vi "EchoSpacing2.vi"() -> ()   [LabVIEW 2016]
uses:
  <vilib>/Analysis/3filter.llb/Filter Passband Type.ctl
  <vilib>/Analysis/NI_AALBase.lvlib
  <vilib>/Analysis/NI_AAL_SigProc.lvlib
  <vilib>/measure/NI_MABase.lvlib
panel:
  out "x/y 2":waveform(dbl)(graph)
  out "output waveform 4":waveform(dbl)(graph)
  out "output waveform 3":waveform(dbl)(graph)
  out "x after average":waveform(dbl)(graph)
  out "output waveform 2":waveform(dbl)(graph)
  out "Change in Speed of Sound":waveform(dbl)(graph)
  out "Phase":waveform(dbl)(graph)={"t0"=timestamp(0 s since 1904-01-01), "dt"=0.01, "Y"=[0.24211856243178442, 0.2979552577953536, 0.11762633618423823, -2.123508525918916, 0.20375659578318772, 0.23633325543017147, 0.10596858427793898, 0.35715128699234333, 0.3077330737862175, 0.29550230623359586, 0.26625637959678994, 0.4264526096514324]}
  out "millisecond timer value":u32=1848068
  out "Array":dbl[](array[numeric])=[0.6752734595800559, 1.1017260692314883, 0.6444600524294382, -1.442367499041461, -0.42475301826616657, 0.660304709391192, -1.2354533445502307, 0.27782180017105296, 1.2450593883598915, -0.8212746442960503, 0.8254110535070931, -0.826966642108493, 0.9668932937884392, -0.35218129117363, -0.35017284449625363, -1.426552428665809, 1.4327256876579455, 0.8973316502630515, 0.47447322742299236, -0.049748678045329967, 0.1127488236132522, -0.9412473014471964]
  out "initialized array":dbl[](array[numeric])
  out "Time Locations":dbl[](array[numeric])=[7.954456871737136e-07, 1.0829944804064152e-06, 1.2197668992928399e-06, 2.066421151225249e-06, 3.3334485136545128e-06, 4.592995774084014e-06, 5.857096715588158e-06, 7.158942345651641e-06, 8.398045018304592e-06, 9.645253296365048e-06, 1.090845897308631e-05, 1.2214698983664545e-05, 1.345038714346347e-05, 1.4701419228763196e-05, 1.4750655022908824e-05, 1.5970949694343346e-05, 1.6041105911005864e-05, 1.7231158138687473e-05, 1.7298645289114775e-05, 1.7383164294270303e-05, 1.8517816256101673e-05, 1.9782665116356317e-05]
  in  "Continuous":bool=TRUE
  in  "Run":bool
  out "output waveform 5":waveform(dbl)(graph)={"t0"=timestamp(0 s since 1904-01-01), "dt"=4e-10, "Y"=array[100000 elements]}
  out "Waveforms":waveform(dbl)[](graph)=[{"t0"=timestamp(0 s since 1904-01-01), "dt"=4e-10, "Y"=array[100000 elements]}, {"t0"=timestamp(2.599999999999738e-07 s since 1904-01-01), "dt"=4e-10, "Y"=array[100000 elements]}]
  out "output waveform":waveform(dbl)(graph)={"t0"=timestamp(2.599999999999738e-07 s since 1904-01-01), "dt"=4e-10, "Y"=array[100000 elements]}
  in  "frequency":dbl=220.0 format="%0.2p"
  in  "Channel (0: Channel 1)":u16(ring) items=["Channel 1", "Channel 2", "Channel 3", "Channel 4", "Math", "Reference 1", "Reference 2", "Reference 3", "Reference 4", "D0", "D1", "D2", "D3", "D4", "D5", "D6", "D7", "D8", "D9", "D10", "D11", "D12", "D13", "D14", "D15", "Amplitude", "Frequency", "Phase", "Normal", "Average", "Maximum Peak Hold", "Minimum Peak Hold"]
  in  "VISA Resource Name":refnum<visa-resource-name>="TCPIP0::10.84.241.74::inst0::INSTR"
  out "Waveform":waveform(dbl)(graph)={"t0"=timestamp(0 s since 1904-01-01), "dt"=4e-10, "Y"=array[100000 elements]}
  in  "threshold":dbl=0.05 format="%0.2f"
  in  "width":i32=150 min=3
  in  "low cutoff freq: fl":dbl=20.0 format="%0.4f"
  out "error":i32
  in  "order":i32=3
  out "total time":u32=34
  # "Single"
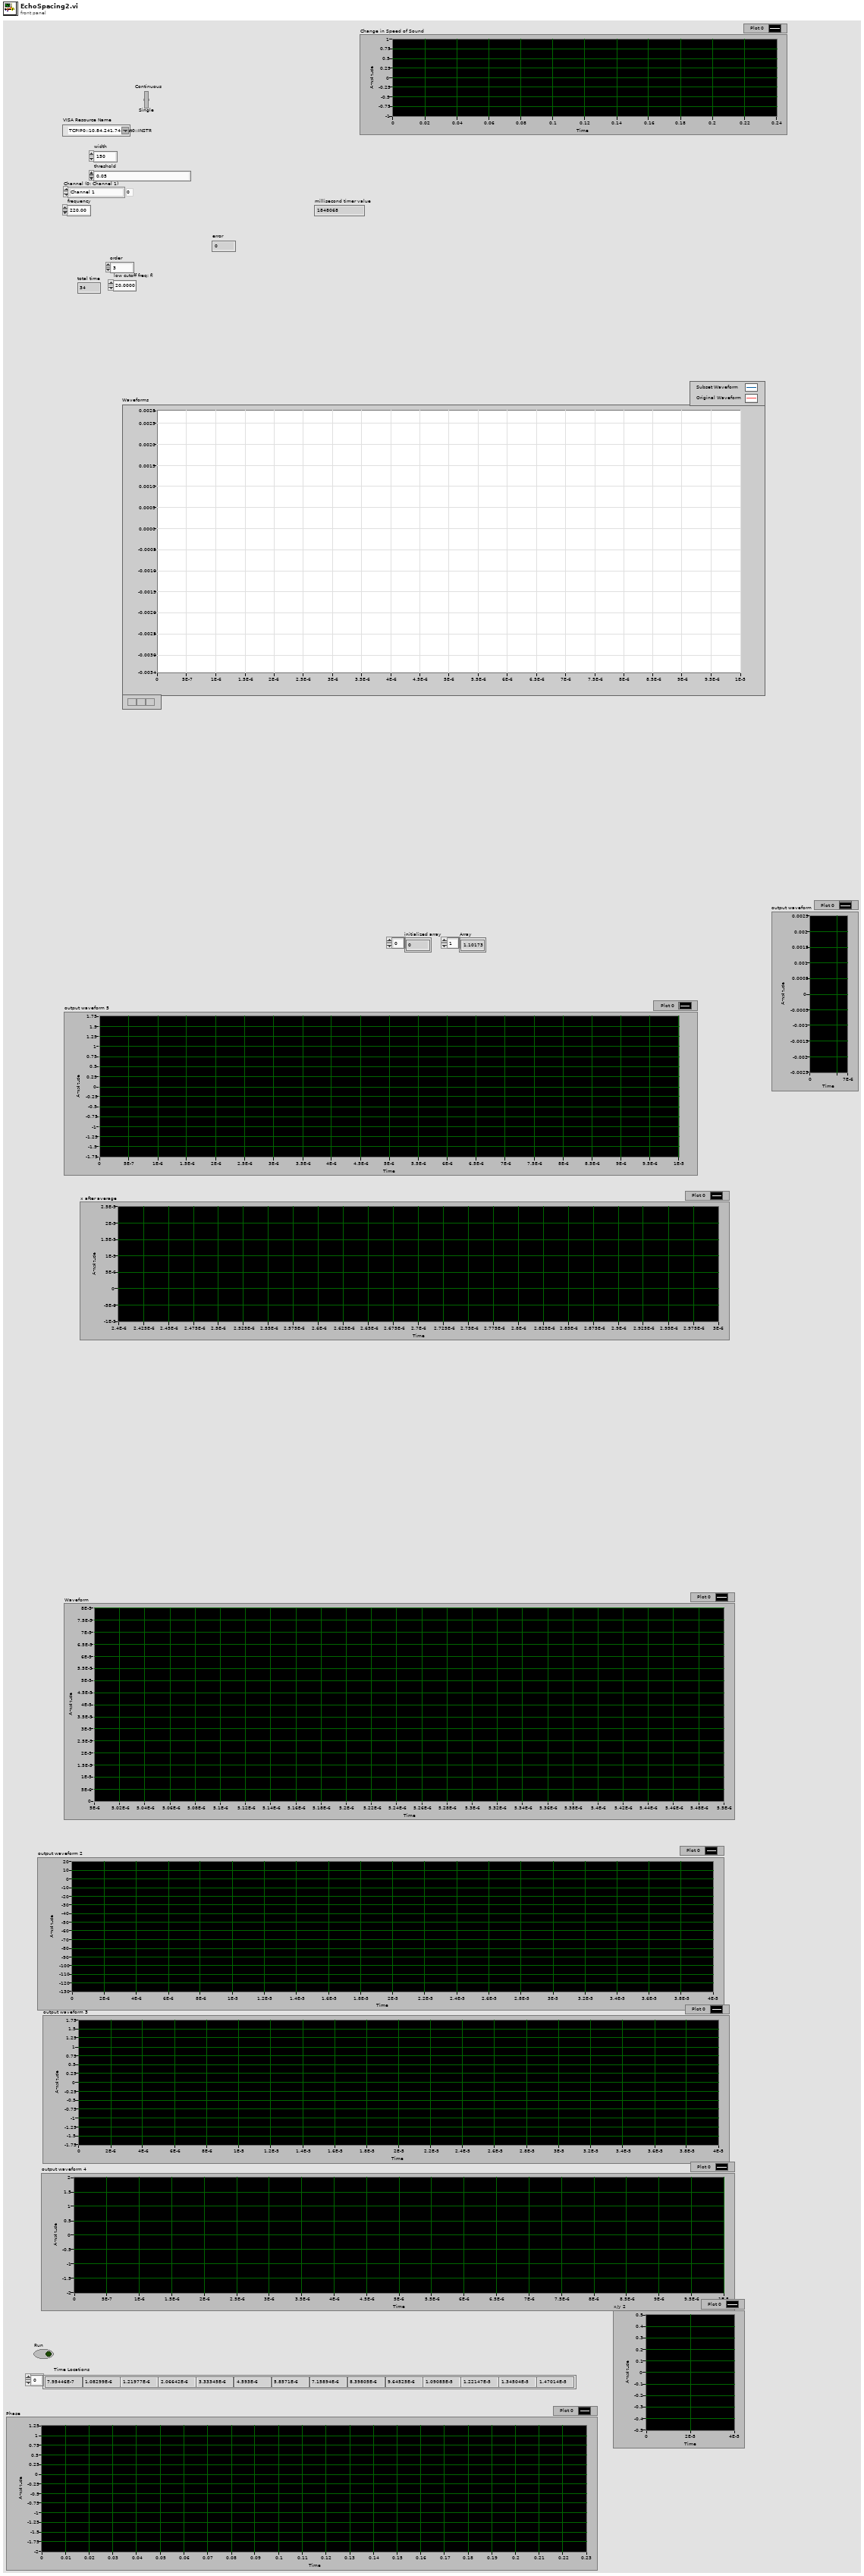
[diagram p1: front panel]
types:
  T1 = typedef "NI_AALBase.lvlib/Filter Passband Type.ctl" = enum32{"Lowpass", "Highpass", "Bandpass", "Bandstop"}
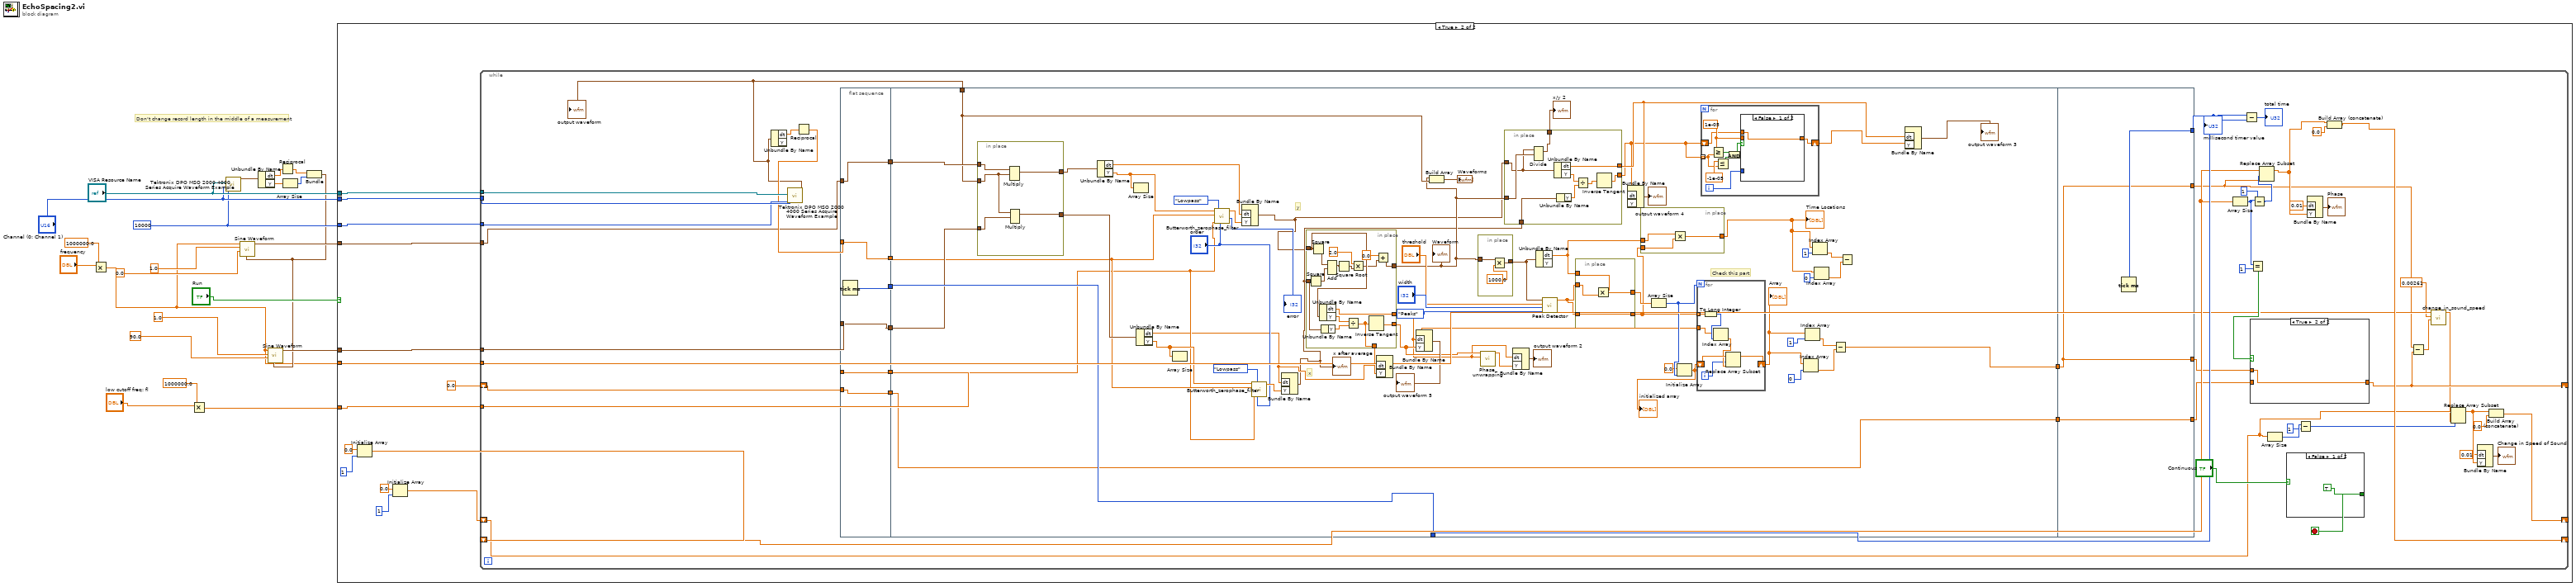
[diagram p0: block diagram]
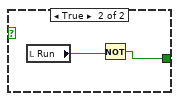
[diagram p4: hidden frame]
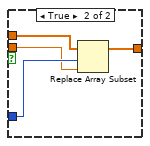
[diagram p5: hidden frame]
diagram:
  w14 = u32 10000 ("Maximum Time (10000ms)")
  # "Don't change record length in the middle of a measurement"
  n1 = Multiply(x="frequency", y=1000000.0) -> (x*y=w1:dbl)
  n2 = Multiply(x="low cutoff freq: fl", y=1000000.0) -> (x*y=w18:dbl)
  n3 = call "Tektronix DPO MSO 2000 4000 Series Acquire Waveform Example.vi"("Maximum Time (10000ms)"=w14, "Channel (0: Channel 1)"="Channel (0: Channel 1)", "VISA Resource Name"="VISA Resource Name") -> ("output waveform"=w7:waveform(dbl))  [unwired: 8 in]
  n4 = Unbundle By Name(w7) -> ("dt"=w5:dbl, "Y"=w6:dbl[])
  n5 = Reciprocal(x=w5) -> (1/x=w4:dbl)
  n6 = Array Size(array=w6) -> (size(s)=w3:i32)
  n7 = Bundle(w4, w3) -> (w2:cluster{dbl, i32})  [unwired: 1 in]
  n8 = call <vilib>:"Sine Waveform.vi"("sampling info"=w2, "phase"=0.0, "amplitude"=1.0, "frequency"=w1) -> ("signal out"=w8:waveform(dbl))  [unwired: 6 in, 1 out]
  n9 = call <vilib>:"Sine Waveform.vi"("sampling info"=w2, "phase"=90.0, "amplitude"=1.0, "frequency"=w1) -> ("signal out"=w11:waveform(dbl))  [unwired: 6 in, 1 out]
  n10 = case shown="True" "Run" {
    tunnel: "VISA Resource Name" -> [_ w36]
    tunnel: "Channel (0: Channel 1)" -> [_ w35]
    tunnel: w14 -> [_ w34]
    tunnel: w18 -> [_ w33]
    tunnel: w11 -> [_ w29]
    tunnel: w8 -> [_ w28]
    tunnel: w1 -> [_ w26]
    frame False {
    }
    frame True {
      n11 = Initialize Array(0.0 ("element"), 1 ("dimension size")) -> (w30:dbl[])
      n12 = Initialize Array(0.0 ("element"), 1 ("dimension size")) -> (w23:dbl[])
      n13 = while {
        tunnel: w36 -> [w79]
        tunnel: w35 -> [w78]
        tunnel: w34 -> [w77]
        tunnel: w33 -> [w75]
        shift-right: [w63] -> _
        shift-left: w30 -> [w70]
        tunnel: w29 -> [w67]
        tunnel: w28 -> [w66]
        shift-right: [w52] -> _
        shift-left: 0.0 -> [w55]
        tunnel: w26 -> [w53]
        shift-right: [w42] -> _
        shift-left: w23 -> [w45]
        stop <- w73 stop-if-true
        n14 = call "Tektronix DPO MSO 2000 4000 Series Acquire Waveform Example.vi"("Maximum Time (10000ms)"=w77, "Channel (0: Channel 1)"=w78, "VISA Resource Name"=w79) -> ("output waveform"=w37:waveform(dbl))  [unwired: 8 in]
        "output waveform" <- w37
        n15 = Unbundle By Name(w37) -> ("dt"=w38:dbl)  [unwired: 1 out]
        n16 = Reciprocal(x=w38) -> (1/x=w76:dbl)
        n17 = flat-sequence {
          tunnel: [w98] -> w87
          tunnel: w76 -> [w97]
          tunnel: [w97] -> w86
          tunnel: [w96] -> w85
          tunnel: w67 -> [w96]
          tunnel: w66 -> [w95]
          tunnel: [w95] -> w84
          tunnel: w75 -> [w94]
          tunnel: [w94] -> w83
          tunnel: w55 -> [w93]
          tunnel: [w93] -> w58
          tunnel: [w155] -> w81
          tunnel: w87 -> [w155]
          tunnel: w86 -> [w137]
          tunnel: w85 -> [w151]
          tunnel: w37 -> [w135]
          tunnel: w84 -> [w152]
          tunnel: w83 -> [w136]
          tunnel: [w99] -> w72
          tunnel: w58 -> [w116]
          tunnel: [w116] -> w57
          tunnel: [w218] -> w82
          tunnel: w72 -> [w216]
          tunnel: [w216] -> w51
          tunnel: w57 -> [w217]
          tunnel: [w217] -> w56
          tunnel: [w216] -> w54
          frame #0 {
            n18 = Tick Count (ms)() -> (millisecond timer value=w98:u32)
          }
          frame #1 {
            # "Check this part"
            # "x"
            # "y"
            n19 = in-place {
              in-place-border: w152 -> [w199]
              in-place-border: w135 -> [w196]
              in-place-border: [w200] -> w153
              in-place-border: w151 -> [w198]
              in-place-border: [w197] -> w150
              n20 = Multiply(1:w196, 2:w199) -> (0:w200:waveform(dbl))  [unwired: 1 in, 1 out]
              n21 = Multiply(1:w198, 2:w196) -> (0:w197:waveform(dbl))  [unwired: 1 in, 1 out]
            }
            n22 = Unbundle By Name(w153) -> ("dt"=w154:dbl, "Y"=w144:dbl[])
            n23 = Array Size(array=w144) -> ()  [unwired: 1 out]
            n24 = Unbundle By Name(w150) -> ("dt"=w110:dbl, "Y"=w138:dbl[])
            n25 = Array Size(array=w138) -> ()  [unwired: 1 out]
            n26 = call "Butterworth_zerophase_filter.vi"("order"="order", "filter type"=Filter_Passband_Type."Lowpass", "low cutoff freq: fl"=w136, "sampling freq: fs"=w137, "X"=w144) -> ("error"=→"error":i32, "Filtered X"=w143:dbl[])  [unwired: 5 in]
            n27 = Bundle By Name("dt"=w154, "Y"=w143) -> (w100:waveform(dbl))  [unwired: 1 in]
            n28 = call "Butterworth_zerophase_filter.vi"("order"="order", "filter type"=Filter_Passband_Type."Lowpass", "low cutoff freq: fl"=w136, "sampling freq: fs"=w137, "X"=w138) -> ("Filtered X"=w140:dbl[])  [unwired: 5 in, 1 out]
            n29 = Bundle By Name("dt"=w110, "Y"=w140) -> (w101:waveform(dbl))  [unwired: 1 in]
            "x after average" <- w101
            n30 = in-place {
              in-place-border: w100 -> [w211]
              in-place-border: w101 -> [w210]
              in-place-border: [w205] -> w109
              in-place-border: [w208] -> w115
              in-place-border: [w209] -> w113
              in-place-border: [w201] -> w111
              n31 = Square(x=w210) -> (x^2=w214:waveform(dbl))
              n32 = Square(x=w211) -> (x^2=w215:waveform(dbl))
              n33 = Unbundle By Name(w211) -> ("dt"=w209:dbl, "Y"=w203:dbl[])
              n34 = Unbundle By Name(w210) -> ("Y"=w202:dbl[])
              n35 = Add(1:w214, 2:w215) -> (0:w213:waveform(dbl))  [unwired: 1 in, 1 out]
              n36 = Square Root(x=w213) -> (sqrt(x)=w212:waveform(dbl))
              n37 = Divide(x=w203, y=w202) -> (x/y=w201:dbl[])
              n38 = Multiply(x=2.0, y=w212) -> (x*y=w206:waveform(dbl))
              n39 = Inverse Tangent(1:w201) -> (0:w208:dbl[])
              n40 = Add(x=0.0, y=w206) -> (x+y=w205:waveform(dbl))
            }
            "Waveform" <- w109
            n41 = Bundle By Name("dt"=w110, "Y"=w111) -> ()  [unwired: 1 in, 1 out]
            n42 = Bundle By Name("dt"=w113, "Y"=w115) -> (→"output waveform 5":waveform(dbl))  [unwired: 1 in]
            n43 = Build Array(w109, w135) -> (→"Waveforms":waveform(dbl)[])
            n44 = in-place {
              in-place-border: w109 -> [w191]
              in-place-border: [w189] -> w133
              n45 = Multiply(x=w191, y=1000.0) -> (x*y=w189:waveform(dbl))
            }
            n46 = call "Phase_unwrapping.vi"("dt"=w113, "phase"=w115) -> ("phase difference"=w114:dbl[])  [unwired: 9 in]
            n47 = in-place {
              in-place-border: w100 -> [w171]
              in-place-border: w109 -> [w172]
              in-place-border: w101 -> [w173]
              in-place-border: [w176] -> w104
              in-place-border: [w175] -> w107
              in-place-border: [w170] -> w105
              n48 = Divide(1:w172, 2:w171) -> (0:w170:waveform(dbl))  [unwired: 1 in, 1 out]
              n49 = Unbundle By Name(w171) -> ("dt"=w175:dbl, "Y"=w178:dbl[])
              n50 = Unbundle By Name(w173) -> ("Y"=w177:dbl[])
              n51 = Divide(x=w178, y=w177) -> (x/y=w174:dbl[])
              n52 = Inverse Tangent(1:w174) -> (0:w176:dbl[])
            }
            "x/y 2" <- w105
            n53 = Bundle By Name("dt"=w113, "Y"=w114) -> (→"output waveform 2":waveform(dbl))  [unwired: 1 in]
            n54 = Unbundle By Name(w133) -> ("dt"=w122:dbl)  [unwired: 1 out]
            n55 = call <vilib>:"Peak Detector.vi"("peaks/valleys"=enum32{"Peaks", "Valleys"}."Peaks", "width"="width", "threshold"="threshold", "X"=w133) -> ("Locations"=w131:dbl[])  [unwired: 3 in, 4 out]
            n56 = in-place {
              in-place-border: w131 -> [w195]
              in-place-border: w122 -> [w194]
              in-place-border: [w193] -> w132
              in-place-border: w131 -> [w192]
              in-place-border: [w192] -> w103
              n57 = Multiply(x=w194, y=w195) -> (x*y=w193:dbl[])
            }
            n58 = Bundle By Name("dt"=w107, "Y"=w104) -> (→"output waveform 4":waveform(dbl))  [unwired: 1 in]
            n59 = in-place {
              in-place-border: w122 -> [w181]
              in-place-border: w103 -> [w180]
              in-place-border: [w179] -> w119
              n60 = Multiply(x=w181, y=w180) -> (x*y=w179:dbl[])
            }
            "Time Locations" <- w119
            n61 = Array Size(array=w132) -> (size(s)=w130:i32)
            n62 = Initialize Array(0.0 ("element"), w130) -> (w128:dbl[])
            "initialized array" <- w128
            n63 = for {
              N: w130 -> [_]
              tunnel: w103 -> [w188] mode=indexing
              tunnel: w115 -> [w186]
              shift-right: [w182] -> w127
              shift-left: w128 -> [w185]
              i -> [w183]
              n64 = To Long Integer(number=w188) -> (32bit integer=w187:i32)
              n65 = Index Array(array=w186, index=w187) -> (element=w184:dbl)
              n66 = Replace Array Subset(array=w185, new element=w184, index=w183) -> (w182:dbl[])
            }
            "Array" <- w127
            n67 = for {
              shift-right: [w156] -> w102
              shift-left: w104 -> [w157]
              tunnel: w104 -> [w163] mode=indexing
              i -> [w159]
              w158 = 1e-05
              n68 = Greater Or Equal?(x=w158, y=w163) -> (x >= y?=w162:bool)
              n69 = Less Or Equal?(x=-1e-05, y=w163) -> (x <= y?=w161:bool)
              n70 = And(x=w162, y=w161) -> (x .and. y?=w160:bool)
              n71 = case shown="False" w160 {
                tunnel: w159 -> [_ w169]
                tunnel: w158 -> [_ w168]
                tunnel: w157 -> [w165 w167]
                tunnel: [w165 w166] -> w156
                frame False {
                }
                frame True {
                  n72 = Replace Array Subset(array=w167, new element=w168, index=w169) -> (w166:dbl[])
                }
              }
            }
            n73 = Index Array(array=w127, index=0) -> (element=w123:dbl)
            n74 = Index Array(array=w127, index=1) -> (element=w124:dbl)
            n75 = Index Array(array=w119, index=1) -> (element=w118:dbl)
            n76 = Index Array(array=w119, index=0) -> (element=w117:dbl)
            n77 = Subtract(x=w124, y=w123) -> (x-y=w99:dbl)
            n78 = Subtract(x=w118, y=w117) -> ()  [unwired: 1 out]
            n79 = Bundle By Name("dt"=w107, "Y"=w102) -> (→"output waveform 3":waveform(dbl))  [unwired: 1 in]
          }
          frame #2 {
            n80 = Tick Count (ms)() -> (millisecond timer value=w218:u32)
          }
        }
        n81 = Array Size(array=w70) -> (size(s)=w61:i32)
        n82 = Subtract(x=w82, y=w81) -> (x-y=→"total time":u32)
        n83 = Equal?(x=w61, y=1) -> (x = y?=w59:bool)
        n84 = case shown="True" w59 {
          tunnel: w56 -> [w88 _]
          tunnel: [w88 w89] -> w52
          tunnel: w54 -> [_ w89]
          frame False {
          }
          frame True {
          }
        }
        n85 = Subtract(x=w61, y=1) -> (x-y=w68:i32)
        n86 = Replace Array Subset(array=w70, new element=w51, index=w68) -> (w65:dbl[])
        n87 = Array Size(array=w45) -> (size(s)=w48:i32)
        n88 = case shown="False" "Continuous" {
          tunnel: [TRUE w91] -> w73
          frame False {
          }
          frame True {
            n89 = local read "Run"() -> (w92:bool)
            n90 = Not(x=w92) -> (.not. x?=w91:bool)
          }
        }
        n91 = Subtract(x=w48, y=1) -> (x-y=w46:i32)
        n92 = Bundle By Name("dt"=0.01, "Y"=w65) -> (→"Phase":waveform(dbl))  [unwired: 1 in]
        n93 = Build Array (concatenate)(w65, 0.0) -> (w63:dbl[])
        n94 = Subtract(x=w51, y=w52) -> (x-y=w50:dbl)
        n95 = call "change_in_sound_speed.vi"("Change in Phase"=w50, "Sample Length"=0.00261, "frequency"=w53) -> ("change in speed"=w44:dbl)  [unwired: 8 in]
        n96 = Replace Array Subset(array=w45, new element=w44, index=w46) -> (w41:dbl[])
        n97 = Bundle By Name("dt"=0.01, "Y"=w41) -> (→"Change in Speed of Sound":waveform(dbl))  [unwired: 1 in]
        n98 = Build Array (concatenate)(w41, 0.0) -> (w42:dbl[])
        "millisecond timer value" <- w82
      }
    }
  }
